vi "Main.vi"() -> ()   [LabVIEW 2020] (continued)
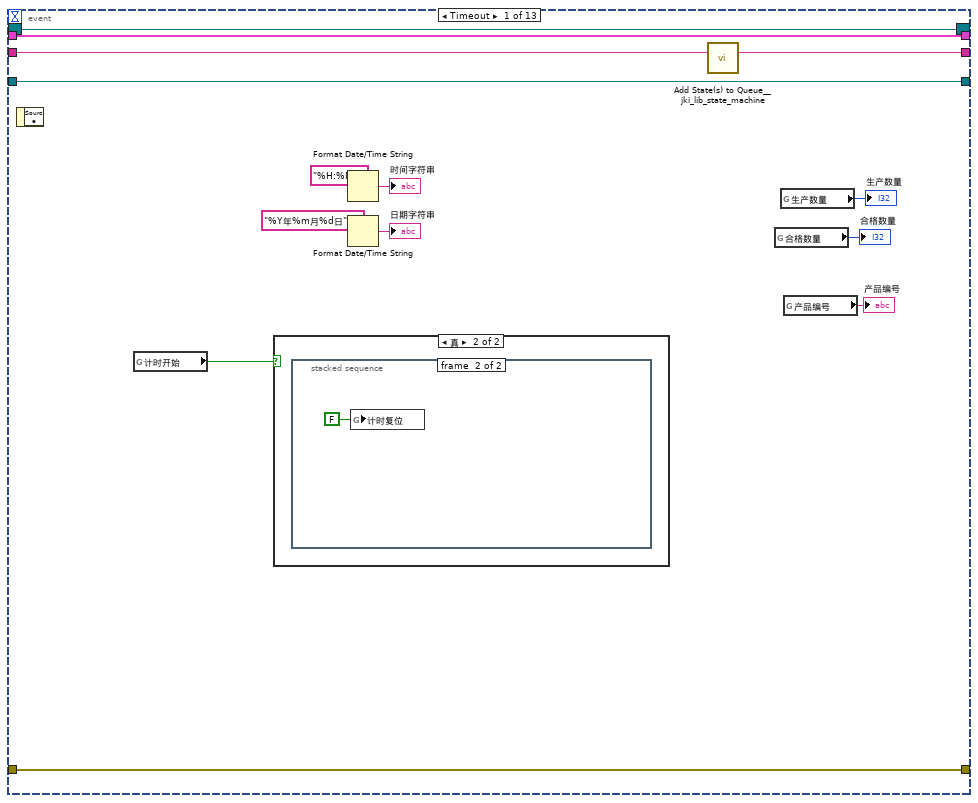
[diagram p2: hidden frame]
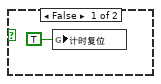
[diagram p3: hidden frame]
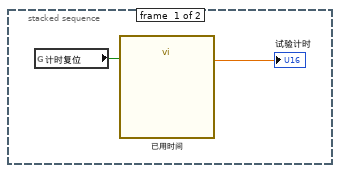
[diagram p4: hidden frame]
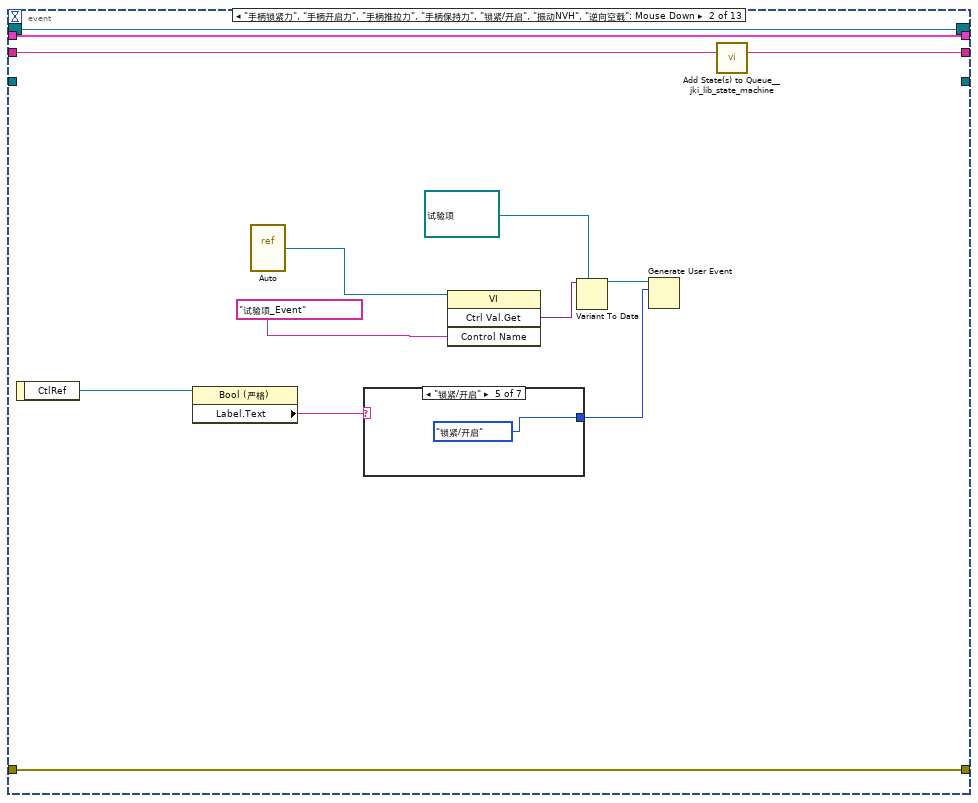
[diagram p5: hidden frame]
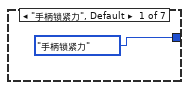
[diagram p6: hidden frame]
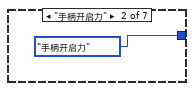
[diagram p7: hidden frame]
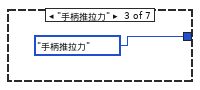
[diagram p8: hidden frame]
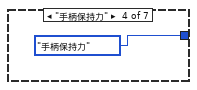
[diagram p9: hidden frame]
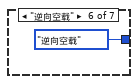
[diagram p10: hidden frame]
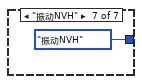
[diagram p11: hidden frame]
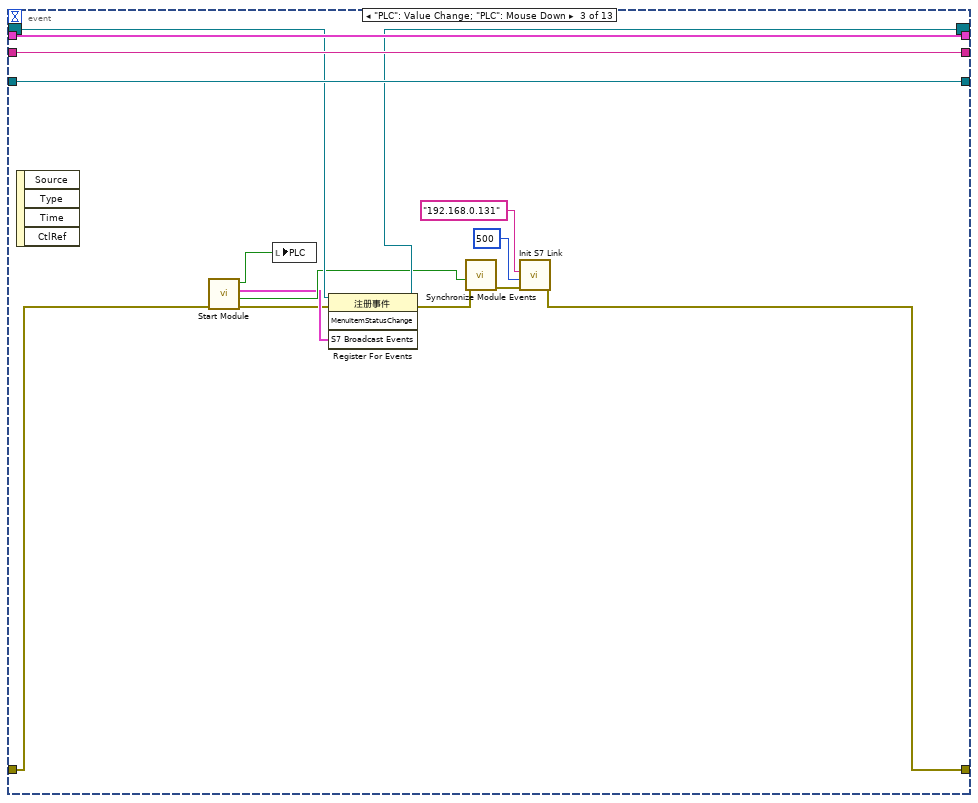
[diagram p12: hidden frame]
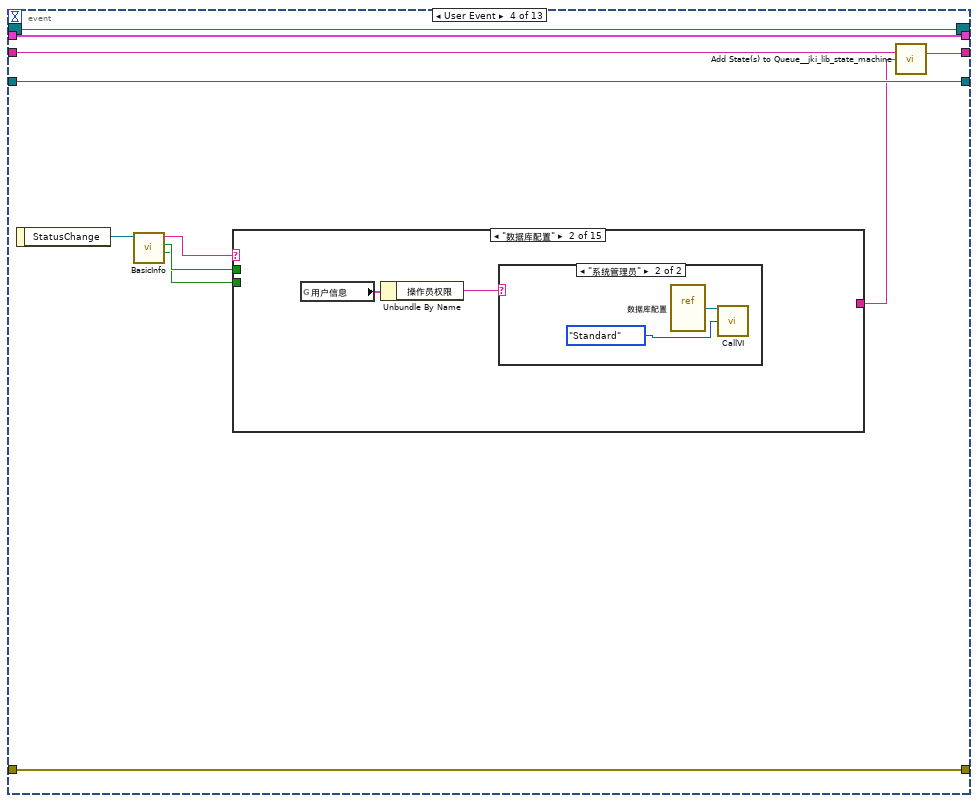
[diagram p13: hidden frame]
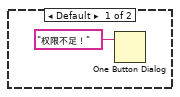
[diagram p15: hidden frame]
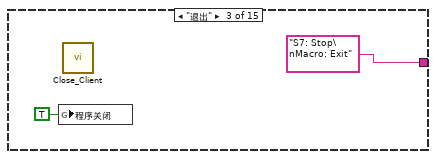
[diagram p16: hidden frame]
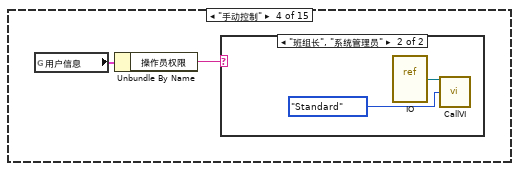
[diagram p17: hidden frame]
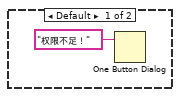
[diagram p18: hidden frame]
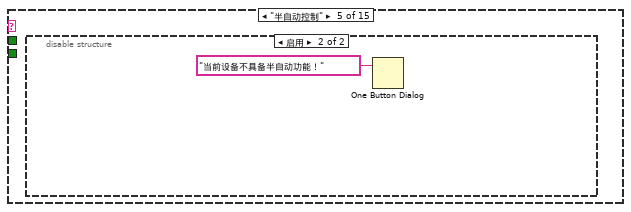
[diagram p19: hidden frame]
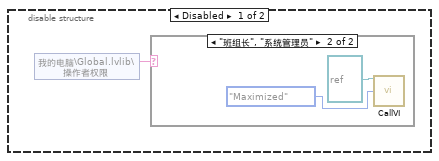
[diagram p20: hidden frame]
                        n119 = invoke class="VI" method="Ctrl Val.Set"(reference=w199, "Control Name"="STEP" ("控件名"), "Value"="退出自动" ("控件名")) -> ()  [unwired: 2 in, 5 out]
                      }
                    }
                  }
                }
              }
              frame Enabled {
              }
            }
            n120 = call <vilib>:"Add State(s) to Queue__jki_lib_state_machine.vi"("State(s) in (\"\")"=w188) -> ("States Out"=w189:string)  [unwired: 14 in]
          }
          event "错误": Mouse Down {
            n121 = event-data() -> ()  [unwired: 1 in, 8 out]
            n122 = vi-ref "报警信息.vi"() -> (w202:refnum<vi>)
            n123 = call "CallVI.vi"("VI引用"=w202, "状态"=T5."Standard") -> ()  [unwired: 12 in, 2 out]
            n124 = call <vilib>:"Add State(s) to Queue__jki_lib_state_machine.vi"("State(s) in (\"\")"=w204) -> ("States Out"=w205:string)  [unwired: 14 in]
          }
          event Panel Close? {
            n125 = event-data() -> ()  [unwired: 1 in, 1 out]
            n126 = global write "Global.vi" "程序关闭"(TRUE ("程序关闭")) -> ()
            n127 = call <vilib>:"Add State(s) to Queue__jki_lib_state_machine.vi"("State(s) in Front (\"\")"="S7: Stop\nMacro: Exit", "State(s) in (\"\")"=w214) -> ("States Out"=w213:string)  [unwired: 13 in]
            n128 = event-data("Discard?"=TRUE) -> ()  [unwired: 1 in, 1 out]
          }
          event "更换产品": Value Change {
            n129 = event-data() -> ("NewVal"=w217:refnum<vi>)  [unwired: 1 in, 5 out]
            n130 = stacked-sequence {
              tunnel: w217 -> [w223]
              tunnel: [w222] -> w215
              frame #0 {
                n131 = stacked-sequence {
                  tunnel: w223 -> [w231 _ _]
                  tunnel: [_ _ "Idle"] -> w222
                  frame #0 {
                    n132 = disable-structure shown="禁用" {
                      disable-tunnel: w231 -> [w233 _]
                      frame Disabled {
                        n133 = control-ref of="子面板"() -> (w232:refnum<vi>)
                        n134 = call "Call_SubPanal.vi"("VI引用句柄"=w233, "SubPnl引用句柄"=w232) -> ()  [unwired: 9 in, 1 out]
                      }
                      frame Enabled {
                      }
                    }
                    n135 = vi-ref "Auto.vi"() -> (w230:refnum<vi>)
                    n136 = global read "Global.vi" "产品型号"() -> (w226:string)
                    n137 = invoke class="VI" method="Ctrl Val.Get"(reference=w230, "Control Name"="标尺_Event" ("控件名")) -> ("Get Control Value Variant"=w229:variant)  [unwired: 2 in, 3 out]
                    n138 = Variant To Data(type=refnum<user-event> refnum ("标尺_Event"), Variant=w229) -> (data=w227:refnum<user-event>, error out=w225:errorcluster)  [unwired: 1 in]
                    n139 = Generate User Event(user event=w227, event data cluster=w226, error in=w225) -> ()  [unwired: 1 in, 2 out]
                    n140 = local write "产品型号"(w226) -> ()
                  }
                  frame #1 {
                    n141 = control-ref of="锁紧/开启"() -> (w234:refnum<vi>)
                    n142 = control-ref of="手柄保持力"() -> (w235:refnum<vi>)
                    n143 = control-ref of="手柄锁紧力"() -> (w236:refnum<vi>)
                    n144 = control-ref of="手柄开启力"() -> (w237:refnum<vi>)
                    n145 = control-ref of="手柄推拉力"() -> (w238:refnum<vi>)
                    n146 = global read "Global.vi" "试验项目"() -> (w241:bool[])
                    n147 = Build Array(w236, w237, w238, w235, w234) -> (w240:refnum<vi>[])
                    n148 = for {
                      tunnel: w240 -> [w245] mode=indexing
                      tunnel: w241 -> [w246] mode=indexing
                      shift-right: [w242] -> _
                      shift-left: 1975 -> [w243]
                      i -> [w244]
                      n149 = case shown="真" w246 {
                        tunnel: w245 -> [w247 w255]
                        tunnel: w244 -> [_ _]
                        tunnel: w243 -> [w249 w252]
                        tunnel: [w249 w250] -> w242
                        frame False {
                          n150 = property class="Bool (严格)"(reference=w247, "Top"=2000) -> ()  [unwired: 1 in, 2 out]
                        }
                        frame True {
                          n151 = Add(x=w252, y=130) -> (x+y=w250:i32)
                          n152 = Bundle(w250, 1250) -> (w253:cluster{i32, i32})  [unwired: 1 in]
                          n153 = property class="Bool (严格)"(reference=w255, "Position"=w253) -> ()  [unwired: 1 in, 2 out]
                        }
                      }
                    }
                  }
                  frame #2 {
                  }
                }
              }
            }
            n154 = call <vilib>:"Add State(s) to Queue__jki_lib_state_machine.vi"("State(s) in Front (\"\")"=w215, "State(s) in (\"\")"=w218) -> ("States Out"=w219:string)  [unwired: 13 in]
          }
          event "Andon": Value Change {
            n155 = event-data() -> ("NewVal"=w261:enum32{"未选择", "缺料报警", "质量报警", "故障报警"})  [unwired: 1 in]
            n156 = case shown="\"未选择\", 默认" w261 {
              tunnel: [enum16{"设备离线", "设备正常", "设备缺料", "设备故障", "质量报警"}."设备正常" ("设备状态") enum16{"设备离线", "设备正常", "设备缺料", "设备故障", "质量报警"}."设备缺料" ("设备状态") enum16{"设备离线", "设备正常", "设备缺料", "设备故障", "质量报警"}."质量报警" ("设备状态") enum16{"设备离线", "设备正常", "设备缺料", "设备故障", "质量报警"}."设备故障" ("设备状态")] -> w259
              frame "未选择", Default {
              }
              frame "缺料报警" {
              }
              frame "质量报警" {
              }
              frame "故障报警" {
              }
            }
            n157 = local read "userName"() -> (w258:string)
            n158 = Bundle By Name(cluster=T6 {"设备名称"="调节机构检测", "操作人员"="", "设备状态"=enum."设备离线", "附加信息"=""} ("设备信息"), "操作人员"=w258, "设备状态"=w259) -> (w257:T6)
            n159 = call "Change_Client.vi"("设备信息"=w257) -> ()  [unwired: 10 in, 1 out]
          }
        }
      }
      frame "---------- Core ----------" {
        n160 = call <vilib>:"Add State(s) to Queue__jki_lib_state_machine.vi"("State(s) in (\"\")"=w275) -> ("States Out"=w274:string)  [unwired: 14 in]
      }
      frame Default {
        w287 = 42 items=["No error", "Argument error", "Memory is full", "Out of zone", "End of file", "File already open", "Generic file I/O error", "File not found", "File permission error", "Disk is full", "Duplicate path", "Too many files open", "System feature not enabled", "Resource file not found", "Cannot add resource", "Resource not found", "Image not found", "Image memory error", "Pen does not exist", "Config type invalid", "Config token not found", "Config parse error", "Config memory error", "Bad external code format", "Bad external code offset", "External code not present", "Null window", "Destroy window error", "Null menu", "Print aborted", "Bad print record", "Print driver error", "Windows error during printing", "Memory error during printing", "Print dialog error", "Generic print error", "Invalid device refnum", "Device not found", "Device parameter error", "Device unit error", "Cannot open device", "Device call aborted", "Generic error", "Cancelled by user", "Object ID too low", "Object ID too high", "Object not in heap", "Unknown heap", "Unknown object (invalid DefProc)", "Unknown object (DefProc not in table)", "Message out of range", "Invalid (null) method", "Unknown message", "Manager call not supported", "Bad address", "Network operation in progress", "Network operation timed out", "Connection is busy", "Network attribute not supported", "Network error", "Address in use", "System out of memory", "Connection aborted", "Connection refused", "Not connected", "Already connected", "Connection closed", "Initialization error (interapplication manager)", "Bad occurrence", "Wait on unbound occurrence handler", "Occurrence queue overflow", "Datalog type conflict", "Unused", "Unrecognized type (interapplication manager)", "Memory corrupt", "Failed to make temporary DLL", "Old CIN version", "Drag socket not found", "Failed to load drop-object", "Failed to register OLE object", "Failed to release OLE object", "Format specifier type mismatch", "Unknown format specifier", "Too few format specifiers", "Too many format specifiers", "Scan failed", "Newer CIN version", "Error converting to variant", "Runtime menu error", "Password tampered", "Variant attribute not found", "Incompatible variant data type", "Event data is not available", "Event Store is not present", "Occurrence is not found", "Event Queue is not created", "Event info is not available", "Refnum passed is NULL", "Error retrieving Class GUID", "Error retrieving CoClass GUID", "Error retrieving TypeLib GUID.", "Bad built application magic bytes.", "Specific driver is different from the specific driver associated with the Logical Name.", "There is no session opened to the class driver.", "Max Error", "MAX - Error with config objects", "MAX - Error loading configuration", "MAX - Group not supported"]
        # "Current State"
        n161 = Format Into String(format string="Software Exception: Unhandled State \"%s\"." ("message"), error in=w283, w278) -> (resulting string=w286:string, error out=w285:errorcluster)  [unwired: 1 in]
        n162 = call <vilib>:"Error Cluster From Error Code.vi"("show call chain? (False)"=TRUE, "error in (no error)"=w285, "error message (\"\")"=w286, "error code (0)"=w287) -> ("error out"=w284:errorcluster)  [unwired: 5 in]
        n163 = call <vilib>:"Add State(s) to Queue__jki_lib_state_machine.vi"("State(s) in (\"\")"=w282) -> ("States Out"=w281:string)  [unwired: 14 in]
      }
      frame "Initialize Core Data" {
        # "originally closed?"
        # "exe?"
        n164 = property class="VI"() -> ("Front Panel.Open"=w298:bool)  [unwired: 2 in, 2 out]
        n165 = property class="App"() -> ("App.Kind"=w297:T7)  [unwired: 2 in, 2 out]
        n166 = control-ref of="Current VI Reference"() -> (w291:refnum<vi>)
        n167 = Not(x=w298) -> (.not. x?=w295:bool)
        n168 = Equal?(x=w297, y=T7."Run Time System" ("Application:Kind")) -> (x = y?=w294:bool)
        n169 = Or(x=w295, y=w294) -> (x .or. y?=w292:bool)
        n170 = Bundle By Name(cluster=w293, "Core.Current VI Reference"=w291, "Core.Close Panel on Exit?"=w292) -> (w300:T9)
        n171 = call <vilib>:"Add State(s) to Queue__jki_lib_state_machine.vi"("State(s) in (\"\")"=w302) -> ("States Out"=w301:string)  [unwired: 14 in]
      }
      frame "Error Handler" {
        n172 = call <vilib>:"General Error Handler.vi"("error in (no error)"=w306) -> ()  [unwired: 10 in, 5 out]
        n173 = call <vilib>:"Add State(s) to Queue__jki_lib_state_machine.vi"("State(s) in Front (\"\")"="/* Post Error States", "State(s) in (\"\")"=w310) -> ("States Out"=w309:string)  [unwired: 13 in]
      }
      frame "Exit" {
        n174 = call <vilib>:"Add State(s) to Queue__jki_lib_state_machine.vi"("State(s) in (\"\")"=w318) -> ("States Out"=w317:string)  [unwired: 14 in]
        n175 = Quit LabVIEW(quit? (T)=TRUE ("退出？(T)")) -> ()
      }
      frame "--------- Library --------" {
        n176 = call <vilib>:"Add State(s) to Queue__jki_lib_state_machine.vi"("State(s) in (\"\")"=w324) -> ("States Out"=w323:string)  [unwired: 14 in]
      }
      frame "S7: Initialize" {
        n177 = property on="PLC" class="Bool (严格)"("Val(Sgnl)"=FALSE ("值(信号)")) -> ()  [unwired: 2 in, 2 out]
      }
      frame "S7: Stop" {
        n178 = call "Stop Module.vi"("error in (no error)"=w333) -> ("error out"=w332:errorcluster)  [unwired: 10 in]
        n179 = call <vilib>:"Add State(s) to Queue__jki_lib_state_machine.vi"("State(s) in (\"\")"=w334) -> ("States Out"=w335:string)  [unwired: 14 in]
      }
      frame "---------- Data ----------" {
        n180 = call <vilib>:"Add State(s) to Queue__jki_lib_state_machine.vi"("State(s) in (\"\")"=w343) -> ("States Out"=w342:string)  [unwired: 14 in]
      }
      frame "Data: Initialize" {
        w349 = T10 {"Current VI Reference"=refnum, "Close Panel on Exit?"=FALSE}  # Core
        w351 = TRUE  # Your Boolean data
        w350 = ""  # Your string data
        n181 = call <userlib>:"Fit VI window to Content__ogtk.vi"("border spacing (2 px)"=1) -> ()  [unwired: 5 in, 2 out]
        n182 = global write "Global.vi" "程序关闭"(FALSE ("程序关闭")) -> ()
        n183 = global write "Global.vi" "计时开始"(FALSE ("计时结束")) -> ()
        n184 = Bundle("Core"=w349, "Your Boolean data"=w351, "Your string data"=w350) -> (w353:T9)  [unwired: 1 in]
        n185 = call <vilib>:"Add State(s) to Queue__jki_lib_state_machine.vi"("State(s) in (\"\")"=w355) -> ("States Out"=w354:string)  [unwired: 14 in]
      }
      frame "Data: Cleanup" {
        n186 = Unbundle By Name(w358) -> ("Core.Current VI Reference"=w361:refnum<vi>)
        n187 = Close Reference(reference=w361, error in (no error)=w360) -> (error out=w359:errorcluster)
        n188 = call <vilib>:"Add State(s) to Queue__jki_lib_state_machine.vi"("State(s) in (\"\")"=w363) -> ("States Out"=w362:string)  [unwired: 14 in]
      }
      frame "---------- UI ----------" {
        # "Do not put any code in this frame.\n(It is a separator no-op. You can make a copy of this frame to create a new UI frame)"
        n189 = call <vilib>:"Add State(s) to Queue__jki_lib_state_machine.vi"("State(s) in (\"\")"=w369) -> ("States Out"=w368:string)  [unwired: 14 in]
      }
      frame "UI: Initialize" {
        n190 = vi-ref "Auto.vi"() -> (w372:refnum<vi>)
        n191 = invoke class="VI" method="Ctrl Val.Set"(reference=w372, "Control Name"="STEP" ("控件名"), "Value"="进入自动" ("控件名")) -> ()  [unwired: 2 in, 5 out]
        n192 = disable-structure shown="启用" {
          disable-tunnel: [w386 _] -> w376
          disable-tunnel: w373 -> [w384 _]
          frame Enabled {
            n193 = vi-ref "Auto.vi"() -> (w385:refnum<vi>)
            n194 = property class="VI"(reference=w385) -> (reference out=w383:refnum<vi>, "FP.State"=w382:T5)  [unwired: 1 in, 1 out]
            n195 = case shown="\"Standard\", 默认" w382 {
              tunnel: w384 -> [w392 w394]
              tunnel: w383 -> [w393 w395]
              tunnel: [w391 w395] -> w380
              tunnel: [w390 w394] -> w381
              frame "Standard", Default {
                n196 = invoke class="VI" method="FP.Close"(reference=w393, error in=w392) -> (reference out=w391:refnum<vi>, error out=w390:errorcluster)  [unwired: 1 in, 1 out]
              }
              frame "Invalid", "Closed" {
              }
            }
            n197 = invoke on="子面板" class="SubPnl" method="Insert VI"(error in=w381, "VI Ref"=w380) -> (error out=w389:errorcluster)  [unwired: 2 in, 3 out]
            n198 = invoke class="VI" method="Run VI"(reference=w380, error in=w389, "Wait until done"=FALSE ("结束前等待"), "Auto Dispose Ref"=TRUE ("自动销毁引用")) -> (error out=w386:errorcluster)  [unwired: 1 in, 4 out]
          }
          frame Disabled {
            n199 = vi-ref "Auto.vi"() -> (w397:refnum<vi>)
            n200 = call "CallVI.vi"("VI引用"=w397, "状态"=T5."Maximized") -> ()  [unwired: 12 in, 2 out]
          }
        }
        n201 = call <vilib>:"Add State(s) to Queue__jki_lib_state_machine.vi"("State(s) in (\"\")"=w379) -> ("States Out"=w378:string)  [unwired: 14 in]
      }
      frame "UI: Init" {
        n202 = stacked-sequence {
          tunnel: w399 -> [_ _ _ _ _]
          frame #0 {
            n203 = property on="上学状态" class="Str"("Text.BGColor"=u32 16777216 ("文本.文本颜色:背景色")) -> ()  [unwired: 2 in, 2 out]
          }
          frame #1 {
            n204 = global write "Global.vi" "程序关闭"(FALSE ("程序关闭")) -> ()
            n205 = control-ref of="锁紧/开启"() -> (w408:refnum<vi>)
            n206 = control-ref of="手柄锁紧力"() -> (w411:refnum<vi>)
            n207 = control-ref of="手柄推拉力"() -> (w409:refnum<vi>)
            n208 = control-ref of="手柄开启力"() -> (w410:refnum<vi>)
            n209 = global write "A180648.vi" "LED-手柄锁紧力"(w411) -> ()
            n210 = global write "A180648.vi" "LED-手柄开启力"(w410) -> ()
            n211 = global write "A180648.vi" "LED-电流特性"(w408) -> ()
            n212 = global write "A180648.vi" "LED-推拉力"(w409) -> ()
            n213 = control-ref of="振动NVH"() -> (w406:refnum<vi>)
            n214 = control-ref of="手柄保持力"() -> (w407:refnum<vi>)
            n215 = global write "A180648.vi" "LED-振动NVH"(w406) -> ()
            n216 = global write "A180648.vi" "LED-保持力"(w407) -> ()
            n217 = control-ref of="上学状态"() -> (w405:refnum<vi>)
            n218 = global write "Global.vi" "上序状态颜色"(w405) -> ()
          }
          frame #2 {
            w421 = 0
            n219 = global read "Global.vi" "上序状态颜色"() -> (w414:refnum<vi>)
            n220 = shared-variable "我的电脑\\Global.lvlib\\总成追溯码"("   " ("工位追溯码")) -> ()  [unwired: 1 in, 1 out]
            n221 = global write "Global.vi" "生产数量"(w421) -> ()
            n222 = global write "Global.vi" "合格数量"(w421) -> ()
            n223 = global read "Global.vi" "用户信息"() -> (w418:T11)
            n224 = global read "Global.vi" "联机模式"() -> (w415:enum16{"单机", "追溯"})
            n225 = property class="Str"(reference=w414, "Value"="" ("值")) -> ()  [unwired: 1 in, 2 out]
            n226 = Unbundle By Name(w418) -> ("用户名"=→"userName":string, "用户权限"=→"userStatus":string)
            n227 = case shown="\"追溯\"" w415 {
              tunnel: ["联网" ("connectionMode") "单机" ("connectionMode")] -> w422
              frame "追溯" {
              }
              frame "单机", Default {
              }
            }
            "connectionMode" <- w422
            "产品型号" <- "" ("产品型号")
          }
          frame #3 {
            n228 = control-ref of="表格控件"() -> (w425:refnum<vi>)
            n229 = control-ref of="提示信息"() -> (w427:refnum<vi>)
            n230 = control-ref of="自动"() -> (w428:refnum<vi>)
            n231 = control-ref of="错误"() -> (w429:refnum<vi>)
            n232 = control-ref of="更换产品"() -> (w426:refnum<vi>)
            n233 = global write "Global.vi" "提示信息"(w427) -> ()
            n234 = global write "Global.vi" "程序自动"(w428) -> ()
            n235 = global write "Global.vi" "报警图标"(w429) -> ()
            n236 = global write "Global.vi" "Result"(w425) -> ()
            n237 = global write "Global.vi" "更换产品"(w426) -> ()
          }
          frame #4 {
            w430 = -2
            n238 = global read "Global.vi" "Result"() -> (w433:refnum<vi>)
            n239 = property class="Tbl"(reference=w433, "Row Headers[]"=string[] [], "Value"=string[][] []) -> ()  [unwired: 1 in, 2 out]
            n240 = Bundle(w430, w430) -> (w431:cluster{i32, i32})  [unwired: 1 in]
            n241 = property class="Tbl"(reference=w433, "Active Cell"=w431, "Cell BG Color"=u32 16777216 ("活动单元格:单元格背景色")) -> ()  [unwired: 1 in, 2 out]
            n242 = call "Start_Client.vi"() -> ()  [unwired: 12 in]
          }
        }
        n243 = call <vilib>:"Add State(s) to Queue__jki_lib_state_machine.vi"("State(s) in (\"\")"=w403) -> ("States Out"=w402:string)  [unwired: 14 in]
      }
      frame "UI: Config" {
        n244 = vi-ref "Config.vi"() -> (w438:refnum<vi>)
        n245 = call "CallVI.vi"("VI引用"=w438, "状态"=T5."Standard") -> ()  [unwired: 12 in, 2 out]
        n246 = call <vilib>:"Add State(s) to Queue__jki_lib_state_machine.vi"("State(s) in (\"\")"=w443) -> ("States Out"=w442:string)  [unwired: 14 in]
      }
      frame "UI: Cursor Set" {
        # "Argument"
        n247 = case shown="\"Idle\", 默认" w446 {
          tunnel: w448 -> [w453 w455]
          tunnel: [w452 w454] -> w447
          frame "Idle", Default {
            n248 = call <vilib>:"Unset Busy.vi"("error in (no error)"=w453) -> ("error out"=w452:errorcluster)  [unwired: 10 in]
          }
          frame "Busy" {
            n249 = call <vilib>:"Set Busy.vi"("error in (no error)"=w455) -> ("error out"=w454:errorcluster)  [unwired: 9 in, 1 out]
          }
        }
        n250 = call <vilib>:"Add State(s) to Queue__jki_lib_state_machine.vi"("State(s) in (\"\")"=w451) -> ("States Out"=w450:string)  [unwired: 14 in]
      }
      frame "UI: Front Panel State" {
        # "Argument"
        n251 = Unbundle By Name(w460) -> ("Core.Current VI Reference"=w459:refnum<vi>)
        n252 = case shown="\"Close\"" w458 {
          tunnel: w462 -> [w468 w481]
          tunnel: [w470 w482] -> w461
          tunnel: w459 -> [w469 w479]
          frame "Open", Default {
            n253 = property class="VI"(reference=w469, error in=w468) -> (reference out=w466:refnum<vi>, error out=w467:errorcluster, "Front Panel.Open"=w465:bool)
            n254 = case shown="假" w465 {
              tunnel: [w473 w476] -> w470
              tunnel: w467 -> [w472 w476]
              tunnel: w466 -> [w471 _]
              frame False {
                n255 = invoke class="VI" method="FP.Open"(reference=w471, error in=w472, "Activate"=TRUE, "State"=T5."Standard") -> (error out=w473:errorcluster)  [unwired: 1 in, 4 out]
              }
              frame True {
              }
            }
          }
          frame "Close" {
            n256 = property class="VI"(reference=w479, error in=w481) -> (reference out=w478:refnum<vi>, error out=w480:errorcluster, "Front Panel.Open"=w477:bool)
            n257 = case shown="真" w477 {
              tunnel: [w483 w486] -> w482
              tunnel: w480 -> [w483 w485]
              tunnel: w478 -> [_ w484]
              frame False {
              }
              frame True {
                n258 = invoke class="VI" method="FP.Close"(reference=w484, error in=w485) -> (error out=w486:errorcluster)  [unwired: 1 in, 2 out]
              }
            }
          }
        }
        n259 = call <vilib>:"Add State(s) to Queue__jki_lib_state_machine.vi"("State(s) in (\"\")"=w464) -> ("States Out"=w463:string)  [unwired: 14 in]
      }
      frame "---------- Macro ----------" {
        n260 = call <vilib>:"Add State(s) to Queue__jki_lib_state_machine.vi"("State(s) in (\"\")"=w492) -> ("States Out"=w491:string)  [unwired: 14 in]
      }
      frame "Macro: Initialize" {
        n261 = call <vilib>:"Add State(s) to Queue__jki_lib_state_machine.vi"("State(s) in Front (\"\")"="Data: Initialize\nInitialize Core Data\nS7: Initialize\nIdle\nUI: Init\nUI: Front Panel State >> Open\nUI: Initialize\nUI: Config", "State(s) in (\"\")"=w499) -> ("States Out"=w498:string)  [unwired: 13 in]
      }
      frame "Macro: Exit" {
        n262 = Unbundle By Name(w508) -> ("Core.Close Panel on Exit?"=w507:bool)
        n263 = Select(t="UI: Front Panel State >> Close", s=w507, f="") -> (s? t:f=w504:string)
        n264 = call <vilib>:"Add State(s) to Queue__jki_lib_state_machine.vi"("State(s) in (\"\")"=w504, "State(s) at Back (\"\")"="Data: Cleanup\nExit") -> ("States Out"=w502:string)  [unwired: 13 in]
        n265 = call <vilib>:"Add State(s) to Queue__jki_lib_state_machine.vi"("State(s) in Front (\"\")"=w502, "State(s) in (\"\")"=w511) -> ("States Out"=w510:string)  [unwired: 13 in]
      }
    }
  }
  n266 = call-dynamic "Cleanup.vi"("MenuStrip in"=w6) -> ()  [unwired: 10 in, 1 out]
